vi "HFRR ADV v042.vi"() -> ()   [LabVIEW 2025] (continued)
  # "Step 3 — Calibration Head"
  # "Place the calibration holder in position and securely tighten the center screw."
  # "Step 4 — Calibration Holder"
  # "Place the calibration holder in position and tighten the two securing screws"
  # "Step 5 — Tare (Spring at Free Length)"
  # "Ensure the spring is at its contact (compressed) length — the micrometer head is in contact. Click Tare Sensor to zero the friction force baseline."
  # "Step 6 — Measure Friction Force"
  # "Run the Actual Test to measure Friction Force."
  # "Step 7 — CALIBRATION RESULT"
  # "Calibration completed successfully. The measured friction force is within the acceptable tolerance range of the factory calibration value."
  # "Calibration failed. The measured friction force differs from the factory calibration value . Please perform the calibration again."
  # "Spring Constant: k = 1.000 N/mm\nSpring force |F| = k Ч d"
  # "Calibrates the sample/bath temperature sensor. \nUsed for test specimen and lubricant temperature measurement."
  # "Calibrates the ambient air temperature sensor. \nUsed for environmental chamber monitoring."
  # "Set B\n60 °C\nHigh-point calibration"
  # "Set A\n0 °C\nIce-point calibration"
  # "Set B\n60 °C\nHigh-point calibration"
  # "Set A\n0 °C\nIce-point calibration"
  # "Select Temperature Sensor"
  # "Choose which temperature sensor you are calibrating. Both use the same two-\npoint procedure: 0 °C (ice-point) and 60 °C (high-point)."
  # "Step 1 — Reference Instrument Setup"
  # "Connect a calibrated reference to the DUT port. This calibration performs two sets: one at 0 °C and one at 60 °C."
  # "Set A\n0 °C\nIce-point calibration"
  # "Set B\n60 °C\nHigh-point calibration"
  # "Allow the temperature bath to stabilise for at least 2 minutes at each set-point before recording the reading."
  # "Step 2 — Set A:  0 °C Calibration"
  # "Connect the  0 °C reference connector. Wait for the temperature to stabilise. Once stable, and click Record Point."
  # "Step 3 — Set B:  60 °C Calibration"
  # "Connect the  60 °C reference connector. Wait for the temperature to stabilise. Once stable, and click Record Point."
  # "Sample Temperature Calibration Complete"
  # "Sample Temperature Calibration PASSED\nMax deviation 0.200 °C — within ±0.5 °C tolerance. Two-point correction applied (0 °C & 60 °C)."
  # "Sample  Temperature Calibration Failed\nmeasured Sample Temperature differs from the factory calibration value"
  # "Step 1 — Reference Instrument Setup"
  # "Connect a calibrated reference to the DUT port. This calibration performs two sets: one at 0 °C and one at 60 °C."
  # "Set A\n0 °C\nIce-point calibration"
  # "Set B\n60 °C\nHigh-point calibration"
  # "Allow the temperature bath to stabilise for at least 2 minutes at each set-point before recording the reading."
  # "Step 2 — Set A:  0 °C Calibration"
  # "Connect the  0 °C reference connector. Wait for the temperature to stabilise. Once stable, and click Record Point."
  # "Step 3 — Set B:  60 °C Calibration"
  # "Connect the  60 °C reference connector. Wait for the temperature to stabilise. Once stable, and click Record Point."
  # "Air Temperature Calibration Complete"
  # "Air Temperature Calibration PASSED\nMax deviation 0.200 °C — within ±0.5 °C tolerance. Two-point correction applied (0 °C & 60 °C)."
  # "Air  Temperature Calibration Failed\nmeasured Sample Temperature differs from the factory calibration value"
  # "System Control Commands\nS;1 - Starts the full automation cycle (Runs Priming-humidify till 70RH sequence first, then switches to Maintenance).\nS;0 - Stops the system immediately and enters Standby mode (Safe State: All actuators OFF).\nM;1 - Skips the priming sequence and jumps directly to Maintenance mode (PID control).\nR;1 - Resets the logic state machine and clears all errors, returning to Standby.\nService Mode (Manual Control)\nX;1 - Enters Manual Service Mode. This disables all automatic logic, sensor safety checks, and timers.\nX;0 - Exits Manual Service Mode and returns to Standby (Safe State).\nActuator Commands (Only work after sending X;1)\nP;[0-255] - Sets the Pump PWM. Note that this is Active Low (0 = Max Flow, 255 = Pump OFF).\nF;I;[0-255] - Sets the Intake Fan speed (0 = OFF, 255 = Max Speed).\nF;O;[0-255] - Sets the Exhaust Fan speed (0 = OFF, 255 = Max Speed).\nD;1 - Turns the Dehumidifier Relay ON.\nD;0 - Turns the Dehumidifier Relay OFF."
  # "%RH"
  # "ISO : WS1.4"
  # "Start test and end test log--- done\nDisable heater ON and Humidity ON during the test --- done\ntemprature and ---done\nhumidity reach log\nauto start run true logic and log\nmanual start log once"
  # "Reference Fluid Information"
  # "Note:\nMake sure to place all images in the folder \"C:\\WinDucom\\im\" before clicking on \"Import Image.\""
  # "NOTE:\nPlace all the images in the path \"C:\\WinDucom\\im\" before clicking on Import Image"
  # "Wear Scar Measurements"
  # "Reference Fluid Information"
  # "Graph :"
types:
  T1 = enum32{"Home", "Dashboard", "Imaging", "Report", "Analysis", "About", "Test Setup", "Advance", "Calibration"}
  T2 = enum32{"HOME", "Test Setup", "Acquire", "Adv Scar", "Adv Scar Report", "Compare Files", "Calibration", "About", "Advance", "Mooha"}
  T3 = enum16{"ASTM D6079", "ISO 12156", "CEC F-096-A-06", "Custom"}
  T4 = enum32{"Dashboard 1", "Dashboard 2", "Dashboard 3"}
  T5 = enum32{"COF", "Friction", "ECR", "Temperature", "Stroke"}
  T6 = enum32{"Coefficient Of Friction", "Air Temperature", "Humidity", "Stroke", "Sample Temperature", "Electrical Contact Resistance", "Frequency", "Air Temp vs Rh"}
  T7 = enum32{"Main", "Stroke", "Friction", "Temperature"}
  T8 = enum32{"Stroke Calibration", "Friction Force Calibration", "Temperature Calibration", "Default"}
  T9 = enum32{"Step 1", "Step 2", "Step 3", "Step 4", "Step 5", "Step 6", "Step 7", "Step 8", "Step 9"}
  T10 = enum32{"Test Progress", "Stroke Points Completed"}
  T11 = enum32{"Page 1", "Page 2", "Page 3", "Page 4", "Page 5", "Page 6"}
  T12 = enum32{"Main", "Step 1", "Step 2", "Step 3", "Step 4", "Air Step 1", "Air Step 2", "Air Step 3", "Air Step 4"}
  T13 = enum32{"Air Temperature", "Sample Temperature", "Default"}
  T14 = enum32{"COMMUNICATION", "CALIBRATION", "Temp Variables", "Camera", "WO 2465 (1)", "WO 2465 (2)", "WO 2465 (3)"}
  T15 = typedef "Auto Start enum.ctl" = enum16{"Init", "Humidity & Temperature On", "Reach point", "Maintain Stage", "Start Stage", "close", "Exit"}
  T16 = typedef "imagedata.ctl" = cluster{"image type":i32, "image depth":i32, "image":u8[], "mask":u8[], "colors":u32[], "Rectangle":cluster{"left":i16, "top":i16, "right":i16, "bottom":i16}}
  T17 = enum32{"HOME", "Test Setup", "Acquire", "Compare Files", "Print Report", "About", "Advance", "Mooha"}
  T18 = cluster{"Read Heave and Surge":string, "Bytes at Heave Port":dbl, "Heave and Surge COM Port:":refnum<visa-resource-name>, "Com Port 2":refnum<visa-resource-name>, "Residual Due":string, "Heave COM Status 2":bool, "Heave COM Status":bool, "Port 2":bool, "Sway PPR":dbl, "Surge PPR":dbl, "Heave PPR":dbl, "Sway Pitch":dbl, "Surge Pitch":dbl, "Heave Pitch":dbl, "Sway Pulses/mm":dbl, "Surge Pulses/mm":dbl, "Heave Pulses/mm":dbl, "inner loop":dbl, "Read Heave and Surge 2":string, "String 36":string, "Write S":bool, "WriteCC1":string[], "Heave COM Loop":i32, "LastCom":string, "EXIT":bool, "Error Heave":errorcluster}
  T19 = enum8{"Enabled", "Disabled", "Disabled and Grayed Out"}
  T20 = cluster{"Read Uno":string, "Bytes at Heave Port":dbl, "UNO COM Port:":refnum<visa-resource-name>, "UNO COM Port: 2":refnum<visa-resource-name>, "Residual Due":string, "UNO COM Status 2":bool, "UNO COM Status":bool, "Port 2":bool, "Sway PPR":dbl, "Surge PPR":dbl, "Heave PPR":dbl, "Sway Pitch":dbl, "Surge Pitch":dbl, "Heave Pitch":dbl, "Sway Pulses/mm":dbl, "Surge Pulses/mm":dbl, "Heave Pulses/mm":dbl, "inner loop":dbl, "Read Heave and Surge 2":string, "String 36":string, "Write S":bool, "WriteCC1":string[], "Heave COM Loop":i32, "LastCom":string, "EXIT":bool, "Error Heave":errorcluster}
  T21 = enum32{"HOME", "Test Setup", "Acquire", "Adv Scar", "Adv Scar Report", "Compare Files", "About", "Advance", "Mooha"}
  T22 = typedef "POST ANALYSIS ENUM.ctl" = enum16{"OPEN EXE", "INIT", "OPEN FILE", "FIT", "DRAW REC", "DRAW LINE", "PAN", "ZOOM IN", "ZOOM OUT", "SET ZOOM", "CLEAR ROI", "GET MEASUREMENTS", "RESIZE MODE", "STREAM START", "STREAM STOP", "SHOW UI", "MINIMIZE UI", "HIDE UI", "CKISE APP", "CLOSE CONNECTION", "SAVE IMAGE", "SET ROI COLOR", "READ", "TCP CHECK", "CLOSE"}
  T23 = typedef "CAMERA LIVE FEED ENUM.ctl" = enum16{"OPEN EXE", "INIT", "READ", "CAMERA CONNECT", "CAMERA START", "CAMERA STOP", "CAMERA GRAY", "CAMERA RGB", "CAMERA MINIMIZE", "CAMERA CLOSE", "CAMERA MODE LIST", "CAMERA MODE SET", "CAMERA RESTORE", "CAMERA SAVE", "CLOSE"}
  T24 = enum16{"Always On", "Always Off", "Off While Running"}
  T25 = enum32{"Home", "Dashboard", "Imaging", "Report", "Analysis", "About", "Test Setup", "Advance"}
  T26 = cluster{"File Name":string, "Test Method":string, "Operator":string, "Fuel Description":string, "Date and time":string}
  T27 = enum32{"Home", "Dashboard", "Imaging", "Report", "Analysis", "About", "Test Setup"}
  T28 = enum32{"HOME", "Test Setup", "Acquire", "Compare Files", "About", "Advance", "Mooha"}
  T29 = typedef "NI_ReportGenerationCore.lvlib/HTML Report Image Alignment.ctl" = enum16{"(default)", "LEFT", "RIGHT", "TOP", "TEXTTOP", "MIDDLE", "ABSMIDDLE", "BASELINE", "BOTTOM", "ABSBOTTOM"}
  T30 = cluster{"y":dbl, "LVDT STROKE DISPLAY":dbl, "y":dbl}
  T31 = enum16{"INIT", "READ", "MANUAL WRITE", "WRITE", "CLOSE", "ERROR INIT"}
diagram:
  w5 = 0.0 ("ch0_filt")
  w7 = -9999999.0 ("max_ch0")
  w8 = 9999999.0 ("min_ch0")
  w19 = FALSE ("Visible")
  w20 = T19."Enabled" ("Disabled")
  w23 = FALSE ("Visible")
  w22 = FALSE ("Humidity Off Command")
  w38 = "" ("USER ID")
  (unwired) T21."HOME" ("Main Tab")
  # "Temperature Continue Air Step 2"
  # "[CH1]    - FF\n[CH2]   - TEMPERATURE\n[CH3]    - Humidity\n[CH4]    - AIR TEMP\n[CH5]\\- Visa Uno\n[CH6] \\- Visa Due\n[CH7]  \\- file path\n[CH8]   - Displacement Gain\n[CHA]   - Stroke Gain\n[CHB]   - Stroke PID Gain\n[CHC]   -Language Selection\n[CHD]   -Power +\n[CHE]   -Power_\n[CHF]   -Heater\n[CHG]   -Humidity Wet\n[CHH]   -Humidity Dry\n[CHI]   -Integral Time \n[CHIJ   -Air intercept\n[CHI]   -Temp Intercept"
  n1 = local write "Cal Password"("" ("Cal Password")) -> ()
  n2 = property on="Auto Start Test" class="Bool (strict)"("Visible"=TRUE) -> ()  [unwired: 2 in, 2 out]
  n3 = property on="FRICVALZ 2" class="Bool (strict)"("DisabledEnum"=w20) -> ()  [unwired: 2 in, 2 out]
  n4 = property on="FRICVALZ 4" class="Bool (strict)"("DisabledEnum"=w20) -> ()  [unwired: 2 in, 2 out]
  n5 = property on="FRICVALZ 3" class="Bool (strict)"("DisabledEnum"=w20) -> ()  [unwired: 2 in, 2 out]
  n6 = property on="About" class="Clust (strict)"("Visible"=FALSE) -> ()  [unwired: 2 in, 2 out]
  n7 = property on="Wrong Password" class="Str"("Visible"=w19) -> ()  [unwired: 2 in, 2 out]
  n8 = property on="Calibration 2" class="TabCtl (strict)"("Visible"=w19) -> ()  [unwired: 2 in, 2 out]
  n9 = local write "Temperature Selection"(T13."Default" ("Temperature Selection")) -> ()
  n10 = flat-sequence {
    tunnel: [w67] -> w4
    tunnel: [w112] -> w30
    tunnel: w4 -> [w107]
    tunnel: [w113] -> w32
    tunnel: w30 -> [w113]
    tunnel: w32 -> [w173]
    tunnel: [w173] -> w31
    tunnel: w31 -> [w204]
    tunnel: [w204] -> w41
    tunnel: w41 -> [w211]
    tunnel: [w217] -> w29
    tunnel: [w205] -> w28
    tunnel: [w259] -> w3
    tunnel: [w258] -> _
    tunnel: w29 -> [w258]
    tunnel: w28 -> [w259]
    frame #0 {
      n11 = call "CLOSE CONNECTION.vi"("error in (no error)"="error in (no error) 2") -> ("error out"=w72:errorcluster)  [unwired: 10 in]
      n12 = call <vilib>:"Clear Errors.vi"("error in (no error)"=w72) -> ("error out"=w71:errorcluster)  [unwired: 5 in, 1 out]
      n13 = disable-structure shown="Enabled" {
        disable-tunnel: w71 -> [w99 _]
        disable-tunnel: [w98 _] -> w70
        frame Enabled {
          n14 = call <userlib>:"Fit VI window to Largest Dec.vi"("error in (no error)"=w99, "border spacing (2 px)"=1) -> ("error out"=w102:errorcluster, "dup VI Ref"=w106:refnum<vi>)  [unwired: 4 in]
          n15 = invoke on="Invoke Node" class="VI" method="FP.Run-Time Position.Maximized"(reference=w106, error in=w102) -> (error out=w103:errorcluster)  [unwired: 2 in, 3 out]
          n16 = call <vilib>:"Clear Errors.vi"("error in (no error)"=w103) -> ("error out"=w105:errorcluster)  [unwired: 5 in, 1 out]
          n17 = control-ref of="This VI"() -> (w97:refnum<vi>)
          n18 = invoke on="Invoke Node" class="VI" method="Default Vals.Reinit All"(reference=w97, error in=w105) -> (reference out=w101:refnum<vi>, error out=w100:errorcluster)  [unwired: 1 in, 1 out]
          n19 = Close Reference(reference=w101, error in (no error)=w100) -> (error out=w98:errorcluster)
        }
        frame Disabled {
        }
      }
      n20 = call "Stall Data Flow.vim"("value in"=w70, "milliseconds to wait"=u32 2000) -> ("value out"=w69:errorcluster)  [unwired: 1 out]
      n21 = call "Read Config.vi"("error in (no error)"=w69) -> ("error out"=w67:errorcluster, "STROKE PARAMETERS"=w78:dbl[], "ADC PARAMETERS"=w79:dbl[], "PID  PARAMETERS"=w80:dbl[], "CALIBRATION PARAMETERS"=w65:string[], "Stroke Calibration"=w77:string)  [unwired: 5 in]
      n22 = Index Array(array=w78) -> (element #1=w95:dbl, element #2=w96:dbl)  [unwired: 2 in]
      n23 = Index Array(array=w65) -> (element #1=w64:string, element #2=w63:string, element #3=w62:string, element #4=w61:string, element #5=w60:string)  [unwired: 5 in]
      n24 = Index Array(array=w79) -> (element #1=w91:dbl, element #2=w92:dbl, element #3=w93:dbl, element #4=w94:dbl, element #5=w59:dbl)  [unwired: 5 in]
      n25 = Index Array(array=w80) -> (element #1=w82:dbl, element #2=w83:dbl, element #3=w84:dbl, element #4=w85:dbl, element #5=w86:dbl, element #6=w87:dbl, element #7=w88:dbl, element #8=w89:dbl, element #9=w90:dbl)  [unwired: 9 in]
      n26 = local write "STROKE FILTER"(w95) -> ()
      n27 = local write "Add up Stroke"(w96) -> ()
      n28 = local write "milliseconds to wait"(w82) -> ()
      n29 = local write "dt"(w83) -> ()
      n30 = local write "kp"(w84) -> ()
      n31 = local write "ki"(w85) -> ()
      n32 = local write "kd"(w86) -> ()
      n33 = local write "max_step_change"(w87) -> ()
      n34 = local write "max_amplitude"(w88) -> ()
      n35 = local write "min_amplitude"(w89) -> ()
      n36 = local write "startup_cmd"(w90) -> ()
      n37 = local write "VREF"(w91) -> ()
      n38 = local write "ADC_Resolution"(w92) -> ()
      n39 = local write "PIEZO_CAL_FACTOR"(w93) -> ()
      n40 = local write "NORMAL_FORCE"(w94) -> ()
      n41 = local write "Machine Serial Number"(w60) -> ()
      n42 = local write "STROKE CALIBRATION"(w64) -> ()
      n43 = local write "FRICTION CALIBRATION"(w63) -> ()
      n44 = local write "TEMPERATURE CALIBRATION"(w62) -> ()
      n45 = Fract/Exp String To Number(string=w61) -> (number=w66:dbl)  [unwired: 3 in, 1 out]
      n46 = local write "FF CAL EXCPTED VALUE"(w59) -> ()
      n47 = Spreadsheet String To Array(delimiter (Tab)=";", format string="", spreadsheet string=w77, array type (2D Dbl)=dbl[] []) -> (array=w81:dbl[])
      n48 = local write "Temperature diff"(w66) -> ()
      n49 = local write "calibration values"(w81) -> ()
    }
    frame #1 {
      n50 = property on="Auto Scar Check" class="Clust (strict)"("Visible"=TRUE) -> ()  [unwired: 2 in, 2 out]
      n51 = property on="Sign In" class="Bool (strict)"("DisabledEnum"=T19."Disabled" ("Disabled")) -> ()  [unwired: 2 in, 2 out]
      n52 = local write "sign in temp"(FALSE ("sign in temp")) -> ()
      n53 = call "dialog box.vi"("Status"="Before starting the test, verify that the microscope cable is connected.", "error in"=w107) -> ("error out"=w112:errorcluster)  [unwired: 8 in]
    }
    frame #2 {
      (unwired) TRUE ("Re-Initialise")
      # "kkkkk"
      # "C:\\Windows\\wndcm_pw_stdED hfrr.txt"
      # "C:\\LAB-IQ NXT"
      # "C:\\LAB-IQ NXT\\wndcm_pw_stdED hfrr.txt"
      # "password file"
      n54 = Current VI's Path() -> (path=w129:path)
      n55 = Strip Path(path=w129) -> (stripped path=w122:path)  [unwired: 1 out]
      n56 = local write "main tab sub"(enum32{"Page 1", "Page 2"}."Page 1" ("main tab sub")) -> ()
      n57 = local write "Main Tab Display"(T4."Dashboard 1" ("Main Tab Display")) -> ()
      n58 = local write "Main Tab"(T2."HOME" ("Main Tab")) -> ()
      n59 = Path To String(path=w122) -> (string=w124:string)
      n60 = Search/Split String(string=w124, search string/char (-)=".exe") -> (match + rest of string=w126:string)  [unwired: 1 in, 2 out]
      n61 = Match True/False String(2:".vi" ("false string"), 3:".exe" ("true string"), 4:w126) -> (0:w123:bool)  [unwired: 1 out]
      n62 = List Folder(path=path "C:/LAB-IQ" ("directory path"), pattern="*.txt") -> (filenames=w135:string[])  [unwired: 2 in, 3 out]
      n63 = case shown="True" w123 {
        tunnel: w122 -> [w144 w146]
        tunnel: [w144 w145] -> w120
        frame False {
        }
        frame True {
          n64 = Strip Path(path=w146) -> (stripped path=w145:path)  [unwired: 1 out]
        }
      }
      n65 = Search 1D Array(1D array=w135, element="wndcm_pw_stdED hfrr.txt") -> (index of element=w138:i32)  [unwired: 1 in]
      n66 = Equal?(x=w138, y=-1) -> (x = y?=w133:bool)
      n67 = Path To String(path=w120) -> (string=→"Gain path":string)
      n68 = case shown="True" w133 {
        frame False {
        }
        frame True {
          n69 = String To Byte Array(string="123\n") -> (unsigned byte array=w151:u8[])
          n70 = Array Size(array=w151) -> (size(s)=w150:i32)
          n71 = for {
            N: w150 -> [_]
            tunnel: w151 -> [w164]
            tunnel: [w161] -> w153 mode=indexing
            tunnel: w150 -> [w156]
            i -> [w154]
            n72 = Decrement(x=w156) -> (x-1=w157:i32)
            n73 = Index Array(array=w164, index=w154) -> (element=w163:u8)
            n74 = Equal?(x=w154, y=w157) -> (x = y?=w158:bool)
            n75 = Number To Decimal String(number=w163) -> (decimal integer string=w162:string)  [unwired: 1 in]
            n76 = Select(t="", s=w158, f="\r") -> (s? t:f=w155:string)
            n77 = Concatenate Strings(w162, w155) -> (w161:string)
          }
          n78 = local read "file path"() -> (w147:path)
          n79 = Concatenate Strings(w153) -> (w149:string)
          n80 = call <vilib>:"Write Characters To File.vi"("append to file? (new file:F)"=FALSE, "character string"=w149, "file path (dialog if empty)"=w147) -> ()  [unwired: 2 in, 1 out]
        }
      }
      n81 = local write "conststatus"(0.0 ("rpm value : 2")) -> ()
      n82 = local write "EVENT LOG"("") -> ()
      n83 = local write "COUNT"(0 ("COUNT")) -> ()
      n84 = local write "clk"(0.0 ("clk")) -> ()
      n85 = local write "Flag"(0.0 ("Flag")) -> ()
      n86 = local write "Lan flag"(0.0 ("Lan flag")) -> ()
      n87 = local write "Com flag"(u32 0 ("Com flag")) -> ()
      n88 = local write "refresh flag"(FALSE ("refresh flag")) -> ()
      "file path" <- path "C:/LAB-IQ/wndcm_pw_stdED hfrr.txt" ("file path")
      "FF buffer" <- dbl[] [] ("FF buffer")
    }
    frame #3 {
      # "C:\\WinDucom\\calibrate WO 2391.dcf"
      n89 = String To Path(string="C:\\LAB-IQ\\Image Calibrate v01.dcf") -> (path=w168:path)
      n90 = String To Path(string="C:\\LAB-IQ\\calibrate WO 2465.dcf") -> (path=w172:path)
      n91 = Open/Create/Replace File "Open File"(file path (use dialog)=w172) -> (refnum out=w171:refnum<file>)  [unwired: 5 in, 2 out]
      n92 = Open/Create/Replace File ("Open File")(file path (use dialog)=w168) -> (refnum out=w167:refnum<file>)  [unwired: 5 in, 2 out]
      n93 = for {
        N: 4 -> [_]
        tunnel: w167 -> [w179]
        i -> [w175]
        n94 = Read from Text File ("Read File")(file (use dialog)=w179) -> (text=w180:string)  [unwired: 3 in, 3 out]
        n95 = String Subset(string=w180, offset (0)=6, length (rest)=10 ("length (rest)")) -> (substring=w176:string)
        n96 = Fract/Exp String To Number(string=w176) -> (number=w174:dbl)  [unwired: 3 in, 1 out]
        n97 = case shown="3" w175 {
          tunnel: w174 -> [w181 w182 _ w183 _]
          frame 0 {
            n98 = local write "5x Gain"(w181) -> ()
          }
          frame 1 {
            n99 = local write "10x Gain"(w182) -> ()
          }
          frame 2 {
          }
          frame 3 {
            n100 = local write "100x gain"(w183) -> ()
          }
          frame 4, Default {
          }
        }
      }
      n101 = for {
        N: 24 -> [_]
        tunnel: w171 -> [w192]
        i -> [w186]
        (unwired) TRUE ("line mode (F)")
        n102 = Read from Text File "Read File"(file (use dialog)=w192) -> (text=w191:string)  [unwired: 3 in, 3 out]
        n103 = Match Pattern(string=w191, regular expression="]") -> (after substring=w189:string)  [unwired: 1 in, 3 out]
        n104 = String Subset(string=w191, offset (0)=5, length (rest)=10 ("length (rest)")) -> (substring=w184:string)
        n105 = Fract/Exp String To Number(string=w184) -> (number=w185:dbl)  [unwired: 3 in, 1 out]
        n106 = Match Pattern(string=w189, regular expression="-") -> (before substring=w187:string)  [unwired: 1 in, 3 out]
        n107 = case shown="18" w186 {
          tunnel: w185 -> [_ _ _ _ _ _ _ _ _ _ w199 _ _ _ _ _ _ _ _ _ _ _ _ _ _]
          tunnel: w187 -> [_ _ _ _ w195 w196 w197 _ _ _ _ _ _ _ _ _ _ _ _ _ w200 _ w201 w202 _]
          frame 0 {
          }
          frame 1 {
          }
          frame 2 {
          }
          frame 3 {
          }
          frame 4 {
            n108 = local write "Com Port 1"(w195) -> ()
          }
          frame 5 {
            n109 = local write "Com Port 2"(w196) -> ()
            n110 = local write "visa due"(w196) -> ()
          }
          frame 6 {
            n111 = String To Path(string=w197) -> (path=w198:path)
            n112 = local write "File Path"(w198) -> ()
          }
          frame 7 {
          }
          frame 8 {
          }
          frame 9 {
          }
          frame 10 {
            n113 = local write "Language Selection"(w199) -> ()
          }
          frame 11 {
          }
          frame 12 {
          }
          frame 13 {
          }
          frame 14 {
          }
          frame 15 {
          }
          frame 16 {
          }
          frame 17 {
          }
          frame 18 {
          }
          frame 21 {
          }
          frame 22 {
            n114 = local write "Com Port 3"(w200) -> ()
          }
          frame 23 {
          }
          frame 19 {
            n115 = local write "C3 :"(w201) -> ()
          }
          frame 20 {
            n116 = local write "Camera Port :"(w202) -> ()
          }
          frame 24, Default {
          }
        }
      }
    }
    frame #4 {
      n117 = Wait (ms)(milliseconds to wait=u32 1000) -> ()  [unwired: 1 out]
    }
    frame #5 {
      w220 = u32 2000 ("milliseconds to wait")
      w247 = u32 2000 ("milliseconds to wait")
      n118 = call "CAMERA LIVE FEED FGV.vi"("Enum - Menu"=CAMERA_LIVE_FEED_ENUM."OPEN EXE", "error in (no error)"=w211) -> ("error out"=w253:errorcluster)  [unwired: 8 in, 1 out]
      n119 = call "IMAGE ANALYSIS.vi"("Enum"=POST_ANALYSIS_ENUM."OPEN EXE", "error in"=w211) -> ("error out"=w208:errorcluster)  [unwired: 8 in, 1 out]
      n120 = call "Stall Data Flow.vim"("value in"=w253, "milliseconds to wait"=w247) -> ("value out"=w251:errorcluster)  [unwired: 1 out]
      n121 = call "Stall Data Flow.vim"("value in"=w208, "milliseconds to wait"=u32 8000) -> ("value out"=w207:errorcluster)  [unwired: 1 out]
      n122 = call "CAMERA LIVE FEED FGV.vi"("Enum - Menu"=CAMERA_LIVE_FEED_ENUM."INIT", "error in (no error)"=w251) -> ("error out"=w249:errorcluster)  [unwired: 8 in, 1 out]
      n123 = call "IMAGE ANALYSIS.vi"("Enum"=POST_ANALYSIS_ENUM."INIT", "error in"=w207) -> ("error out"=w205:errorcluster)  [unwired: 8 in, 1 out]
      n124 = case shown="Error .." w249 {
        selector: w249 -> [w254 _]
        tunnel: [w254 _] -> w248
        frame No Error {
        }
        frame Error {
          n125 = One Button Dialog(message="Camera initialization error.\nPlease Restart the software") -> ()  [unwired: 1 in, 1 out]
        }
      }
      n126 = property on="Camera Port :" class="CmbBox"() -> ("Strings[]"=w245:string[], "Value"=w246:string)  [unwired: 2 in, 2 out]
      n127 = Search 1D Array(1D array=w245, element=w246) -> (index of element=w244:i32)  [unwired: 1 in]
      n128 = Type Cast(type=30, x=w244) -> (*(type *) &x=w242:i32)
      n129 = call "Stall Data Flow.vim"("value in"=w248, "milliseconds to wait"=w247) -> ("value out"=w224:errorcluster)  [unwired: 1 out]
      n130 = Add(x=w242, y=48) -> (x+y=w223:i32)
      n131 = call "CAMERA LIVE FEED FGV.vi"("Enum - Menu"=CAMERA_LIVE_FEED_ENUM."CAMERA CONNECT", "error in (no error)"=w224, "CAMERA PORT"=w223) -> ("error out"=w233:errorcluster)  [unwired: 7 in, 1 out]
      n132 = call "Stall Data Flow.vim"("value in"=w233, "milliseconds to wait"=u32 5000) -> ("value out"=w234:errorcluster)  [unwired: 1 out]
      n133 = call "CAMERA LIVE FEED FGV.vi"("Enum - Menu"=CAMERA_LIVE_FEED_ENUM."CAMERA MODE LIST", "error in (no error)"=w234) -> ("error out"=w236:errorcluster)  [unwired: 8 in, 1 out]
      n134 = call "Stall Data Flow.vim"("value in"=w236, "milliseconds to wait"=w220) -> ("value out"=w235:errorcluster)  [unwired: 1 out]
      n135 = call "CAMERA LIVE FEED FGV.vi"("Enum - Menu"=CAMERA_LIVE_FEED_ENUM."READ", "error in (no error)"=w235) -> ("error out"=w222:errorcluster, "data out"=→"Camera List":string)  [unwired: 8 in]
      n136 = Type Cast(type=30, x=0) -> (*(type *) &x=w216:i32)
      n137 = call "Stall Data Flow.vim"("value in"=w222, "milliseconds to wait"=w220) -> ("value out"=w221:errorcluster)  [unwired: 1 out]
      n138 = Add(x=w216, y=48) -> (x+y=w214:i32)
      n139 = call "CAMERA LIVE FEED FGV.vi"("Enum - Menu"=CAMERA_LIVE_FEED_ENUM."CAMERA MODE SET", "error in (no error)"=w221, "CAMERA MODE"=w214) -> ("error out"=w218:errorcluster)  [unwired: 7 in, 1 out]
      n140 = call "Stall Data Flow.vim"("value in"=w218, "milliseconds to wait"=u32 2000) -> ("value out"=w238:errorcluster)  [unwired: 1 out]
      n141 = call "CAMERA LIVE FEED FGV.vi"("Enum - Menu"=CAMERA_LIVE_FEED_ENUM."CAMERA START", "error in (no error)"=w238) -> ("error out"=w239:errorcluster)  [unwired: 8 in, 1 out]
      n142 = call "Stall Data Flow.vim"("value in"=w239, "milliseconds to wait"=u32 1000) -> ("value out"=w240:errorcluster)  [unwired: 1 out]
      n143 = call "CAMERA LIVE FEED FGV.vi"("Enum - Menu"=CAMERA_LIVE_FEED_ENUM."CAMERA MINIMIZE", "error in (no error)"=w240) -> ("error out"=w217:errorcluster)  [unwired: 8 in, 1 out]
    }
    frame #6 {
      n144 = case shown="No Error" w258 {
        frame No Error {
          n145 = property on="Auto Scar Check" class="Clust (strict)"("Visible"=FALSE) -> ()  [unwired: 2 in, 2 out]
        }
        frame Error {
        }
      }
      n146 = property on="Sign In" class="Bool (strict)"("DisabledEnum"=T19."Enabled" ("Disabled")) -> ()  [unwired: 2 in, 2 out]
      n147 = local write "sign in temp"(TRUE ("sign in temp")) -> ()
    }
  }
  n148 = local write "Calibration Selection"(T8."Default" ("Calibration Selection")) -> ()
  n149 = local write "SCAR MEASURMENT"(enum32{"Auto Scar", "Manual Scar"}."Manual Scar" ("SCAR MEASURMENT")) -> ()
  n150 = local write "Temperature Off Command"(w22) -> ()
  n151 = local write "Main Dashboard Buttons"(T1."Home" ("Main Dashboard Buttons")) -> ()
  n152 = local write "Humidity Off Command"(w22) -> ()
  n153 = local write "CAMERA ROI MIN TEMP"(w22) -> ()
  n154 = local write "TEST FILE NAM,E SAVED"(w22) -> ()
  n155 = local write "LIVE FEED MIN TEMP"(w22) -> ()
  n156 = local write "SCAR MEASURMENT"(enum32{"Auto Scar", "Manual Scar"}."Manual Scar" ("SCAR MEASURMENT")) -> ()
  n157 = local write "Auto stop temp"(w23) -> ()
  n158 = local write "main tab sub"(enum32{"Page 1", "Page 2"}."Page 1" ("main tab sub")) -> ()
  n159 = while {
    stop <- w273 stop-if-true
    n160 = local read "Ambient Temperature"() -> (w271:dbl)
    n161 = local read "Sample Temperature"() -> (w270:dbl)
    n162 = Wait (ms)(milliseconds to wait=u32 200) -> ()  [unwired: 1 out]
    n163 = local write "Sensor value"(w271) -> ()
    n164 = local write "Sensor value"(w271) -> ()
    n165 = local write "Sensor value"(w270) -> ()
    n166 = local write "Sensor value"(w270) -> ()
    n167 = local write "Temperature — Live (Set A: 0 °C)"(w271) -> ()
    n168 = local write "Temperature — Live (Set A: 60 °C)"(w271) -> ()
    n169 = local write "Temperature — Live (Set A: 60 °C)"(w270) -> ()
    n170 = local write "Temperature — Live (Set A: 0 °C)"(w270) -> ()
    n171 = case shown="True" "Save Button" {
      selector: "Save Button" -> [_ w327]
      frame False {
      }
      frame True {
        n172 = Not(x=w327) -> (.not. x?=w326:bool)
        n173 = local read "Temperature diff"() -> (w323:dbl)
        n174 = local read "Machine Serial Number"() -> (w312:string)
        n175 = local read "milliseconds to wait"() -> (w359:u32)
        n176 = local write "Save Button"(w326) -> ()
        n177 = local read "max_step_change"() -> (w364:dbl)
        n178 = local read "FF CAL EXCPTED VALUE"() -> (w310:dbl)
        n179 = local read "max_amplitude"() -> (w365:dbl)
        n180 = local read "min_amplitude"() -> (w366:dbl)
        n181 = local read "PIEZO_CAL_FACTOR"() -> (w370:dbl)
        n182 = local read "startup_cmd"() -> (w367:dbl)
        n183 = local read "NORMAL_FORCE"() -> (w371:dbl)
        n184 = local read "ADC_Resolution"() -> (w369:dbl)
        n185 = local read "kp"() -> (w361:dbl)
        n186 = local read "kd"() -> (w363:dbl)
        n187 = local read "calibration values"() -> (w374:dbl[])
        n188 = local read "dt"() -> (w360:dbl)
        n189 = local read "ki"() -> (w362:dbl)
        n190 = local read "STROKE FILTER"() -> (w372:i32)
        n191 = local read "Add up Stroke"() -> (w373:dbl)
        n192 = Number To Fractional String(number=w323) -> (F-format string=w322:string)  [unwired: 3 in]
        n193 = local read "VREF"() -> (w368:dbl)
        n194 = Insert Into Array(array=dbl[] [], new element #1=w359, new element #2=w360, new element #3=w361, new element #4=w362, new element #5=w363, new element #6=w364, new element #7=w365, new element #8=w366, new element #9=w367) -> (w375:dbl[])  [unwired: 1 in]
        n195 = Insert Into Array(array=dbl[] [], new element #1=w368, new element #2=w369, new element #3=w370, new element #4=w371, new element #5=w310) -> (w376:dbl[])  [unwired: 1 in]
        n196 = Array To Spreadsheet String(delimiter (Tab)=";", array=w374, 3:"" ("format string")) -> (spreadsheet string=w378:string)
        n197 = Insert Into Array(array=dbl[] [], new element #1=w372, new element #2=w373) -> (w377:dbl[])  [unwired: 1 in]
        n198 = Insert Into Array(array=string[] [], new element #1="STROKE CALIBRATION", new element #2="FRICTION CALIBRATION", new element #3="TEMPERATURE CALIBRATION", new element #4=w322, new element #5=w312) -> (w324:string[])  [unwired: 1 in]
        n199 = call "Write Config.vi"("Stroke Calibration"=w378, "CALIBRATION PARAMETERS"=w324, "STROKE PARAMETERS"=w377, "ADC PARAMETERS"=w376, "PID  PARAMETERS"=w375) -> ("error out"=w357:errorcluster)  [unwired: 6 in]
        n200 = call "Stall Data Flow.vim"("value in"=w357, "milliseconds to wait"=u32 2000) -> ("value out"=w358:errorcluster)  [unwired: 1 out]
        n201 = call "Read Config.vi"("error in (no error)"=w358) -> ("STROKE PARAMETERS"=w355:dbl[], "ADC PARAMETERS"=w354:dbl[], "PID  PARAMETERS"=w353:dbl[], "CALIBRATION PARAMETERS"=w318:string[], "Stroke Calibration"=w356:string)  [unwired: 5 in, 1 out]
        n202 = Index Array(array=w353) -> (element #1=w351:dbl, element #2=w350:dbl, element #3=w349:dbl, element #4=w348:dbl, element #5=w347:dbl, element #6=w346:dbl, element #7=w345:dbl, element #8=w344:dbl, element #9=w343:dbl)  [unwired: 9 in]
        n203 = Index Array(array=w354) -> (element #1=w342:dbl, element #2=w341:dbl, element #3=w340:dbl, element #4=w339:dbl, element #5=w309:dbl)  [unwired: 5 in]
        n204 = Index Array(array=w355) -> (element #1=w338:dbl, element #2=w337:dbl)  [unwired: 3 in, 1 out]
        n205 = Index Array(array=w318) -> (element #1=w315:string, element #2=w314:string, element #3=w313:string, element #4=w317:string, element #5=w311:string)  [unwired: 5 in]
        n206 = Spreadsheet String To Array(delimiter (Tab)=";", format string="", spreadsheet string=w356, array type (2D Dbl)=dbl[] []) -> (array=w352:dbl[])
        n207 = local write "STROKE CALIBRATION"(w315) -> ()
        n208 = local write "FRICTION CALIBRATION"(w314) -> ()
        n209 = local write "TEMPERATURE CALIBRATION"(w313) -> ()
        n210 = Fract/Exp String To Number(string=w317) -> (number=w316:dbl)  [unwired: 3 in, 1 out]
        n211 = local write "Machine Serial Number"(w311) -> ()
        n212 = local write "STROKE FILTER"(w338) -> ()
        n213 = local write "Add up Stroke"(w337) -> ()
        n214 = local write "VREF"(w342) -> ()
        n215 = local write "ADC_Resolution"(w341) -> ()
        n216 = local write "PIEZO_CAL_FACTOR"(w340) -> ()
        n217 = local write "NORMAL_FORCE"(w339) -> ()
        n218 = local write "FF CAL EXCPTED VALUE"(w309) -> ()
        n219 = local write "calibration values"(w352) -> ()
        n220 = local write "milliseconds to wait"(w351) -> ()
        n221 = local write "dt"(w350) -> ()
        n222 = local write "kp"(w349) -> ()
        n223 = local write "ki"(w348) -> ()
        n224 = local write "kd"(w347) -> ()
        n225 = local write "max_step_change"(w346) -> ()
        n226 = local write "max_amplitude"(w345) -> ()
        n227 = local write "min_amplitude"(w344) -> ()
        n228 = local write "startup_cmd"(w343) -> ()
        n229 = local write "Temperature diff"(w316) -> ()
      }
    }
    n230 = local read "USER ID"() -> (w268:string)
    n231 = local read "run test Calibration"() -> (w266:bool)
    n232 = disable-structure shown="Enabled" {
      disable-tunnel: [w280 w291] -> w267
      frame Disabled {
        n233 = local read "Point 1 - 0.2 mm"() -> (w290:bool)
        n234 = local read "Point 2 - 0.4 mm"() -> (w289:bool)
        n235 = local read "Point 3 - 0.6 mm"() -> (w288:bool)
        n236 = local read "Point 4 - 0.8 mm"() -> (w287:bool)
        n237 = local read "Point 5 - 1.0 mm"() -> (w286:bool)
        n238 = local read "Point 6 - 1.2 mm"() -> (w285:bool)
        n239 = And(x=w290, y=w289) -> (x .and. y?=w284:bool)
        n240 = And(x=w288, y=w287) -> (x .and. y?=w283:bool)
        n241 = And(x=w286, y=w285) -> (x .and. y?=w281:bool)
        n242 = And(x=w284, y=w283) -> (x .and. y?=w282:bool)
        n243 = And(x=w282, y=w281) -> (x .and. y?=w280:bool)
      }
      frame Enabled {
        n244 = local read "Point 5 - 1.0 mm"() -> (w291:bool)
      }
    }
    n245 = local read "START TEMP"() -> (w265:bool)
    n246 = local write "tested by 2"(w268) -> ()
    n247 = And(x=w265, y=w266) -> (x .and. y?=w264:bool)
    n248 = case shown="True" w264 {
      frame False {
        w292 = TRUE ("PAUSE")
        n249 = call "ELAPSED TIMER VI - Calibration.vi"("RESET"=w292, "PAUSE"=w292) -> ()  [unwired: 7 in, 3 out]
      }
      frame True {
        w295 = FALSE ("PAUSE")
        n250 = call "ELAPSED TIMER VI - Calibration.vi"("TARGET"=60.0, "RESET"=w295, "PAUSE"=w295) -> ("ELAPSED INDICATION"=w293:bool)  [unwired: 6 in, 2 out]
        n251 = case shown="True" w293 {
          frame False {
            n252 = local write "Friction Force Calibration Result Tab"(enum32{"Calibration Results", "Page 2"}."Calibration Results" ("Friction Force Calibration Result Tab")) -> ()
            n253 = property on="Friction Force Calibration Result Tab" class="TabCtl (strict)"("Visible"=TRUE) -> ()  [unwired: 2 in, 2 out]
          }
          frame True {
            n254 = stacked-sequence {
              frame #0 {
                n255 = local read "Friction"() -> (→"Friction cal":dbl)
                n256 = local write "START TEMP"(FALSE ("START TEMP")) -> ()
              }
              frame #1 {
                n257 = Wait (ms)(milliseconds to wait=u32 1500) -> ()  [unwired: 1 out]
              }
              frame #2 {
                n258 = local write "Due Write"("VC;0") -> ()
              }
              frame #3 {
                n259 = Wait (ms)(milliseconds to wait=u32 1500) -> ()  [unwired: 1 out]
              }
              frame #4 {
                n260 = local write "Due Write"("VC;0") -> ()
              }
              frame #5 {
                n261 = property on="Friction Force Calibration Result Tab" class="TabCtl (strict)"("Visible"=TRUE) -> ()  [unwired: 2 in, 2 out]
              }
            }
          }
        }
      }
    }
    n262 = local read "Friction cal"() -> (w263:dbl)
    n263 = case shown="False" w267 {
      frame False {
        n264 = property on="Accept & Save" class="Bool (strict)"("DisabledEnum"=T19."Disabled" ("Disabled")) -> ()  [unwired: 2 in, 2 out]
        n265 = property on="Tab Control 5" class="TabCtl (strict)"("Value"=enum32{"OK", "NG"}."NG" ("Tab Control 5")) -> ()  [unwired: 2 in, 2 out]
      }
      frame True {
        n266 = property on="Accept & Save" class="Bool (strict)"("DisabledEnum"=T19."Enabled" ("Disabled")) -> ()  [unwired: 2 in, 2 out]
        n267 = property on="Tab Control 5" class="TabCtl (strict)"("Value"=enum32{"OK", "NG"}."OK" ("Tab Control 5")) -> ()  [unwired: 2 in, 2 out]
      }
    }
    n268 = Greater Or Equal?(x=w263, y="FF CAL EXCPTED VALUE") -> (x >= y?=w261:bool)
    n269 = case shown="False" w261 {
      selector: w261 -> [w274 w277]
      frame False {
        n270 = local write "FF PASS"(w274) -> ()
        n271 = local write "Friction Force result Tab"(enum32{"OK", "NG"}."NG" ("Friction Force result Tab")) -> ()
        n272 = property on="Accept & Save FF" class="Bool (strict)"("DisabledEnum"=T19."Disabled" ("Disabled")) -> ()  [unwired: 2 in, 2 out]
      }
      frame True {
        n273 = local write "Friction Force result Tab"(enum32{"OK", "NG"}."OK" ("Friction Force result Tab")) -> ()
        n274 = property on="Accept & Save FF" class="Bool (strict)"("DisabledEnum"=T19."Enabled" ("Disabled")) -> ()  [unwired: 2 in, 2 out]
        "FF PASS" <- w277
      }
    }
    n275 = local read "Quit"() -> (w273:bool)
  }
  n276 = local write "USERNAME"(w38) -> ()
  n277 = local write "Main Tab"(T2."HOME" ("Main Tab")) -> ()
  n278 = local write "USER ID"(w38) -> ()
  n279 = property on="Auto Scar Check  2" class="Clust (strict)"("Visible"=w23) -> (error out=w26:errorcluster)  [unwired: 2 in, 1 out]
  n280 = property on="Quit" class="Bool (strict)"("Value"=FALSE ("Quit")) -> (error out=w40:errorcluster)  [unwired: 2 in, 1 out]
  n281 = while {
    stop <- w379 stop-if-true
    n282 = event shown="[45] \"FF BACK\", \"FF BACK 2\", \"FF BACK 3\", \"FF BACK 4\", \"FF BACK 5\", \"FF BACK 6\", \"Accept & Save FF\": Value Change" {
      selector: _ -> [_ _ _ _ _ _ _ _ _ _ _ _ _ _ _ _ _ _ _ _ _ _ _ _ _ _ _ _ _ _ _ _ _ _ _ _ _ _ _ _ _ _ _ _ _ _ _ _ _ _ _ _ _ _ _ _]
      dyn-events: _ -> [_ _ _ _ _ _ _ _ _ _ _ _ _ _ _ _ _ _ _ _ _ _ _ _ _ _ _ _ _ _ _ _ _ _ _ _ _ _ _ _ _ _ _ _ _ _ _ _ _ _ _ _ _ _ _ _]
      timeout: 100 -> [_ _ _ _ _ _ _ _ _ _ _ _ _ _ _ _ _ _ _ _ _ _ _ _ _ _ _ _ _ _ _ _ _ _ _ _ _ _ _ _ _ _ _ _ _ _ _ _ _ _ _ _ _ _ _ _]
      tunnel: [FALSE FALSE FALSE _ FALSE _ _ _ _ _ _ _ _ _ _ _ _ _ _ _ _ _ _ _ _ _ _ _ _ _ _ _ _ _ _ _ _ _ _ _ _ _ _ _ _ _ _ _ _ _ _ _ _ _ _ TRUE] -> w379
      event Timeout {
        n283 = event-data() -> ()  [unwired: 1 in, 3 out]
        n284 = disable-structure shown="Disabled" {
          frame Disabled {
            n285 = local read "Auto Start Test"() -> (w393:bool)
            n286 = local read "RUN"() -> (w394:bool)
            n287 = Or(x=w394, y=w393) -> (x .or. y?=w392:bool)
            n288 = case shown="True" w392 {
              frame False {
                w395 = TRUE ("PAUSE")
                n289 = call "ELAPSED TIMER VI - abort test.vi"("RESET"=w395, "PAUSE"=w395) -> ()  [unwired: 7 in, 3 out]
              }
              frame True {
                n290 = local read "Stroke 2"() -> (w400:dbl)
                n291 = local read "FF 3"() -> (w402:dbl)
                n292 = Equal?(x=w400, y=0.95 ("Stroke 2")) -> (x = y?=w397:bool)
                n293 = Equal?(x=w402, y=0.0 ("FF 3")) -> (x = y?=w398:bool)
                n294 = Or(x=w398, y=w397) -> (x .or. y?=w396:bool)
                n295 = case shown="True" w396 {
                  selector: w396 -> [_ w407]
                  frame False {
                    w403 = TRUE ("PAUSE")
                    n296 = call "ELAPSED TIMER VI - abort test.vi"("RESET"=w403, "PAUSE"=w403) -> ()  [unwired: 7 in, 3 out]